vi "Get Wrap Value v2.vi"(9 "SLM Param In":T1={"Error"={"status"=FALSE, "code"=0, "source"=""}, "References"={"Main VI"=refnum, "SLM VI"=refnum}, "Directories"={"Root Directory"=path "C:/Documents and Settings/tg273/My Documents/LabView VIs/Yale SLM/Yale v2/Mode Matrices", "Output Directory"=path "C:/Documents and Settings/tg273/My Documents/LabView VIs/Yale SLM/Yale v2/Mode Matrices"}, "Holo size"=504, "X pos"=-3, "Y pos"=-40, "Mode Coeffs"=[[2.0, 0.0], [3.0, 18.0], [4.0, 0.0], [11.0, 0.0], [22.0, 0.0], [37.0, 0.0], [5.0, 0.0], [6.0, 0.0], [7.0, 0.0], [8.0, 0.0], [9.0, 0.0], [10.0, 0.0]], "Wrap Value"=197, "Lambda (nm)"=750.0, "NA"=1.4, "Base Name"="", "Win Num"=2, "SLM SN"="0600535", "Holo Image Name"="0600535", "Matrix Name"="Unit Matrix.csv", "Mode Matrix"=array36x36[1296 elements], "Flatness"=array600x792[475200 elements], "STED Phase"=array504x504[254016 elements], "Ab Corr"=array504x504[254016 elements], "Holo Image"="remote image 00000000298188F4", "Holo Position"={-3.0, -40.0, 3840.0, 504.0}, "Apply Flatness\ncorr.?"=TRUE, "Max Wavelength (nm)"=750.0, "Min Wavelength (nm)"=750.0, "Vortex Rotation"=-3, "Top Hat Radius"=1.4, "SLM ID Num"="0600535", "Max Zernike Modes"=-3, "Screen Width"=2, "Ab Corr VI"={"AC VI Ref"=refnum, "# Modes"=2, "Mode Array"=[[4.0, 0.0, 0.0, 1.0, 0.0], [11.0, 0.75, 0.0, 1.0, 0.0], [22.0, 0.1, 0.0, 1.0, 0.0], [37.0, 0.0, 0.0, 1.0, 0.0], [7.0, 0.15, 0.0, 1.0, 0.0], [8.0, 0.1, 0.0, 1.0, 0.0], [5.0, 0.05, 0.0, 1.0, 0.0], [6.0, 0.0, 0.0, 1.0, 0.0], [9.0, 0.0, 0.0, 1.0, 0.0], [10.0, 0.0, 0.0, 1.0, 0.0], [2.0, 0.0, 0.0, 1.0, 0.0], [3.0, -18.3, 0.0, 1.0, 0.0]], "Apply Corr?"=TRUE, "Step Size"=0.3, "# Steps  "=11, "Resolution"=0.2, "FOV (um)"=12.0, "Metric Images"=[], "Metric Values"=[], "S"=[120.26, 128.5, 131.1, 136.15, 138.3, 148.05, 149.99, 150.02, 147.88, 152.65, 152.69, 150.56, 144.92, 143.08, 146.19, 140.15, 134.69, 125.47, 117.35, 108.32], "I"=[], "M"=[], "Coeff Steps"=[120.26, 128.5, 131.1, 136.15, 138.3, 148.05, 149.99, 150.02, 147.88, 152.65, 152.69, 150.56, 144.92, 143.08, 146.19, 140.15, 134.69, 125.47, 117.35, 108.32], "Mode Loop"={"Mode"=0, "Metric"=0, "Loop Index"=0}}} {"Vortex Rotation" format="%#_3g"; "Min Wavelength (nm)" format="%#_3g"; "Max Wavelength (nm)" format="%#_3g"; "Mode Matrix" format="%0.3f"; "Wrap Value" format="%#_3g"}) -> (1 "SLM Param Out":T1={"Error"={"status"=FALSE, "code"=0, "source"=""}, "References"={"Main VI"=refnum, "SLM VI"=refnum}, "Directories"={"Root Directory"=path "C:/Documents and Settings/tg273/My Documents/LabView VIs/Yale SLM/Yale v2/Mode Matrices", "Output Directory"=path "C:/Documents and Settings/tg273/My Documents/LabView VIs/Yale SLM/Yale v2/Mode Matrices"}, "Holo size"=504, "X pos"=-3, "Y pos"=-40, "Mode Coeffs"=[[2.0, 0.0], [3.0, 18.0], [4.0, 0.0], [11.0, 0.0], [22.0, 0.0], [37.0, 0.0], [5.0, 0.0], [6.0, 0.0], [7.0, 0.0], [8.0, 0.0], [9.0, 0.0], [10.0, 0.0]], "Wrap Value"=197, "Lambda (nm)"=750.0, "NA"=1.4, "Base Name"="", "Win Num"=2, "SLM SN"="0600535", "Holo Image Name"="0600535", "Matrix Name"="Unit Matrix.csv", "Mode Matrix"=array36x36[1296 elements], "Flatness"=array600x792[475200 elements], "STED Phase"=array504x504[254016 elements], "Ab Corr"=array504x504[254016 elements], "Holo Image"="remote image 00000000298188F4", "Holo Position"={-3.0, -40.0, 3840.0, 504.0}, "Apply Flatness\ncorr.?"=TRUE, "Max Wavelength (nm)"=750.0, "Min Wavelength (nm)"=750.0, "Vortex Rotation"=-3, "Top Hat Radius"=1.4, "SLM ID Num"="0600535", "Max Zernike Modes"=-3, "Screen Width"=2, "Ab Corr VI"={"AC VI Ref"=refnum, "# Modes"=2, "Mode Array"=[[4.0, 0.0, 0.0, 1.0, 0.0], [11.0, 0.75, 0.0, 1.0, 0.0], [22.0, 0.1, 0.0, 1.0, 0.0], [37.0, 0.0, 0.0, 1.0, 0.0], [7.0, 0.15, 0.0, 1.0, 0.0], [8.0, 0.1, 0.0, 1.0, 0.0], [5.0, 0.05, 0.0, 1.0, 0.0], [6.0, 0.0, 0.0, 1.0, 0.0], [9.0, 0.0, 0.0, 1.0, 0.0], [10.0, 0.0, 0.0, 1.0, 0.0], [2.0, 0.0, 0.0, 1.0, 0.0], [3.0, -18.3, 0.0, 1.0, 0.0]], "Apply Corr?"=TRUE, "Step Size"=0.3, "# Steps  "=11, "Resolution"=0.2, "FOV (um)"=12.0, "Metric Images"=[], "Metric Values"=[], "S"=[120.26, 128.5, 131.1, 136.15, 138.3, 148.05, 149.99, 150.02, 147.88, 152.65, 152.69, 150.56, 144.92, 143.08, 146.19, 140.15, 134.69, 125.47, 117.35, 108.32], "I"=[], "M"=[], "Coeff Steps"=[120.26, 128.5, 131.1, 136.15, 138.3, 148.05, 149.99, 150.02, 147.88, 152.65, 152.69, 150.56, 144.92, 143.08, 146.19, 140.15, 134.69, 125.47, 117.35, 108.32], "Mode Loop"={"Mode"=0, "Metric"=0, "Loop Index"=0}}} {"Vortex Rotation" format="%#_3g"; "Min Wavelength (nm)" format="%#_3g"; "Max Wavelength (nm)" format="%#_3g"; "Mode Matrix" format="%0.3f"; "Wrap Value" format="%#_3g"})   [LabVIEW 2014]
uses:
  TypeDefs/SLM Parameters.ctl
  <vilib>/vision/Image Controls.llb/IMAQ Image.ctl
types:
  T1 = typedef "SLM Parameters.ctl" = cluster{"Error":errorcluster, "References":cluster{"Main VI":refnum<vi>, "SLM VI":refnum<vi>}, "Directories":cluster{"Root Directory":path, "Output Directory":path}, "Holo size":u16, "X pos":i16, "Y pos":i16, "Mode Coeffs":dbl[][], "Wrap Value":i32, "Lambda (nm)":dbl, "NA":dbl, "Base Name":string, "Win Num":i32, "SLM SN":string, "Holo Image Name":string, "Matrix Name":string, "Mode Matrix":dbl[][], "Flatness":u8[][], "STED Phase":dbl[][], "Ab Corr":dbl[][], "Holo Image":T2, "Holo Position":cluster{dbl, dbl, dbl, dbl}, "Apply Flatness\ncorr.?":bool, "Max Wavelength (nm)":dbl, "Min Wavelength (nm)":dbl, "Vortex Rotation":i16, "Top Hat Radius":dbl, "SLM ID Num":string, "Max Zernike Modes":i16, "Screen Width":i32, "Ab Corr VI":cluster{"AC VI Ref":refnum<vi>, "# Modes":i32, "Mode Array":dbl[][], "Apply Corr?":bool, "Step Size":dbl, "# Steps  ":u16, "Resolution":dbl, "FOV (um)":dbl, "Metric Images":dbl[][][][], "Metric Values":dbl[][], "S":dbl[], "I":dbl[], "M":dbl[], "Coeff Steps":dbl[], "Mode Loop":cluster{"Mode":i8, "Metric":i8, "Loop Index":i8}}}
  T2 = typedef "IMAQ Image.ctl" = refnum<image>
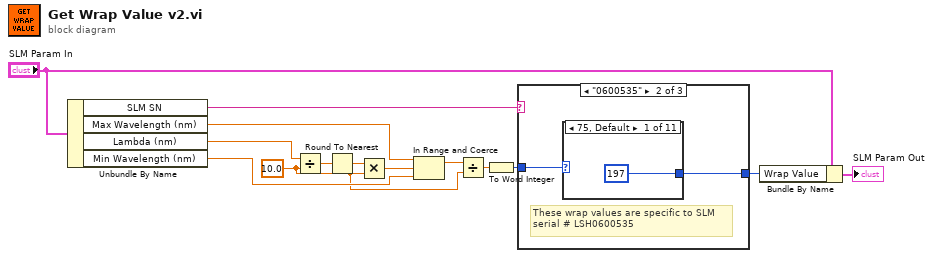
[diagram p0: block diagram]
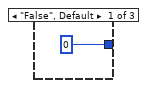
[diagram p2: hidden frame]
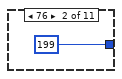
[diagram p3: hidden frame]
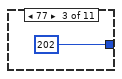
[diagram p4: hidden frame]
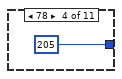
[diagram p5: hidden frame]
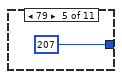
[diagram p6: hidden frame]
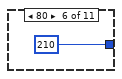
[diagram p7: hidden frame]
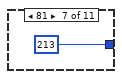
[diagram p8: hidden frame]
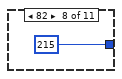
[diagram p9: hidden frame]
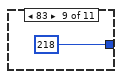
[diagram p10: hidden frame]
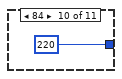
[diagram p11: hidden frame]
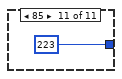
[diagram p12: hidden frame]
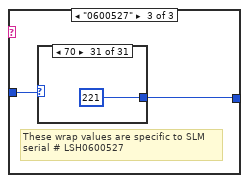
[diagram p13: hidden frame]
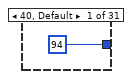
[diagram p14: hidden frame]
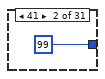
[diagram p15: hidden frame]
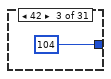
[diagram p16: hidden frame]
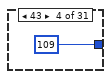
[diagram p17: hidden frame]
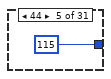
[diagram p18: hidden frame]
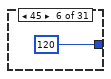
[diagram p19: hidden frame]
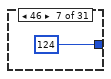
[diagram p20: hidden frame]
diagram:
  w2 = 10.0 ("y")
  n1 = Unbundle By Name("SLM Param In") -> ("SLM SN"=w13:string, "Max Wavelength (nm)"=w10:dbl, "Lambda (nm)"=w1:dbl, "Min Wavelength (nm)"=w9:dbl)
  n2 = Divide(x=w1, y=w2) -> (x/y=w14:dbl)
  n3 = Round To Nearest(number=w14) -> (nearest integer value=w11:dbl)
  n4 = Multiply(x=w11, y=w2) -> (x*y=w12:dbl)
  n5 = In Range and Coerce(upper limit=w10, x=w12, lower limit=w9) -> (coerced(x)=w4:dbl)  [unwired: 1 out]
  n6 = Divide(x=w4, y=w2) -> (x/y=w3:dbl)
  n7 = To Word Integer(number=w3) -> (16bit integer=w5:i16)
  n8 = case shown="\"0600535\"" w13 {
    tunnel: w5 -> [_ w17 w30]
    tunnel: [0 w16 w29] -> w6
    frame "False", Default {
    }
    frame "0600535" {
      # "These wrap values are specific to SLM\nserial # LSH0600535"
      n9 = case shown="75, Default" w17 {
        tunnel: [197 ("wrap val") 199 ("wrap val") 202 ("wrap val") 205 ("wrap val") 207 ("wrap val") 210 ("wrap val") 213 ("wrap val") 215 ("wrap val") 218 ("wrap val") 220 ("wrap val") 223 ("wrap val")] -> w16
        frame 75, Default {
        }
        frame 76 {
        }
        frame 77 {
        }
        frame 78 {
        }
        frame 79 {
        }
        frame 80 {
        }
        frame 81 {
        }
        frame 82 {
        }
        frame 83 {
        }
        frame 84 {
        }
        frame 85 {
        }
      }
    }
    frame "0600527" {
      # "These wrap values are specific to SLM\nserial # LSH0600527"
      n10 = case shown="70" w30 {
        tunnel: [94 ("wrap val") 99 ("wrap val") 104 ("wrap val") 109 ("wrap val") 115 ("wrap val") 120 ("wrap val") 124 ("wrap val") 129 ("wrap val") 134 ("wrap val") 138 ("wrap val") 143 ("wrap val") 147 ("wrap val") 151 ("wrap val") 155 ("wrap val") 159 ("wrap val") 163 ("wrap val") 167 ("wrap val") 170 ("wrap val") 174 ("wrap val") 178 ("wrap val") 182 ("wrap val") 185 ("wrap val") 189 ("wrap val") 193 ("wrap val") 197 ("wrap val") 201 ("wrap val") 204 ("wrap val") 208 ("wrap val") 213 ("wrap val") 217 ("wrap val") 221 ("wrap val")] -> w29
        frame 40, Default {
        }
        frame 41 {
        }
        frame 42 {
        }
        frame 43 {
        }
        frame 44 {
        }
        frame 45 {
        }
        frame 46 {
        }
        frame 47 {
        }
        frame 48 {
        }
        frame 49 {
        }
        frame 50 {
        }
        frame 51 {
        }
        frame 52 {
        }
        frame 53 {
        }
        frame 54 {
        }
        frame 55 {
        }
        frame 56 {
        }
        frame 57 {
        }
        frame 58 {
        }
        frame 59 {
        }
        frame 60 {
        }
        frame 61 {
        }
        frame 62 {
        }
        frame 63 {
        }
        frame 64 {
        }
        frame 65 {
        }
        frame 66 {
        }
        frame 67 {
        }
        frame 68 {
        }
        frame 69 {
        }
        frame 70 {
        }
      }
    }
  }
  n11 = Bundle By Name(cluster="SLM Param In", "Wrap Value"=w6) -> (→"SLM Param Out":T1)
